vi "UHR-Fleezers Control (host) - 10.6.vi"() -> ()   [LabVIEW 2010] (continued)
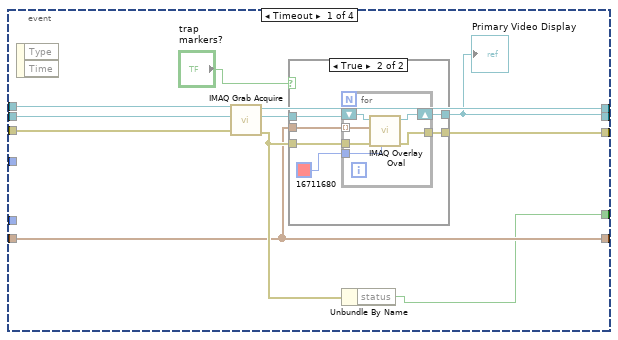
[diagram p2: hidden frame]
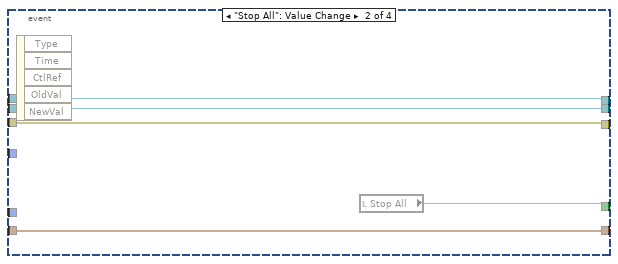
[diagram p4: hidden frame]
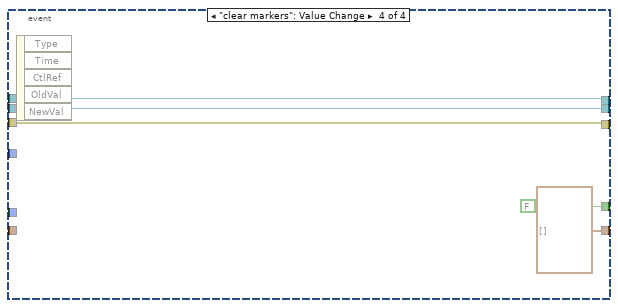
[diagram p6: hidden frame]
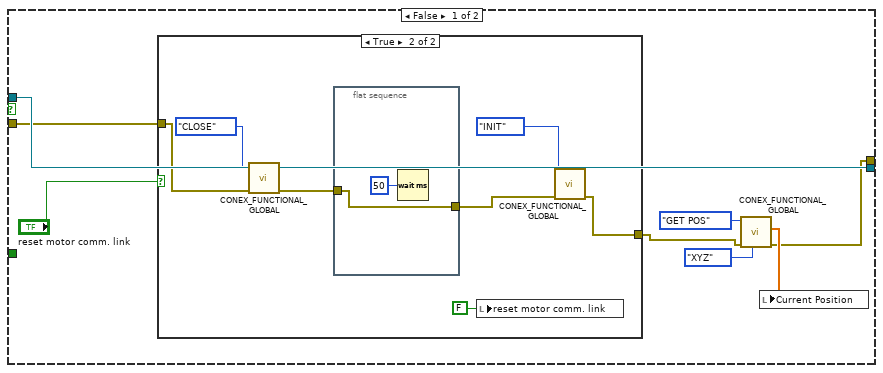
[diagram p8: hidden frame]
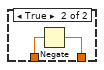
[diagram p12: hidden frame]
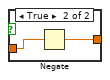
[diagram p13: hidden frame]
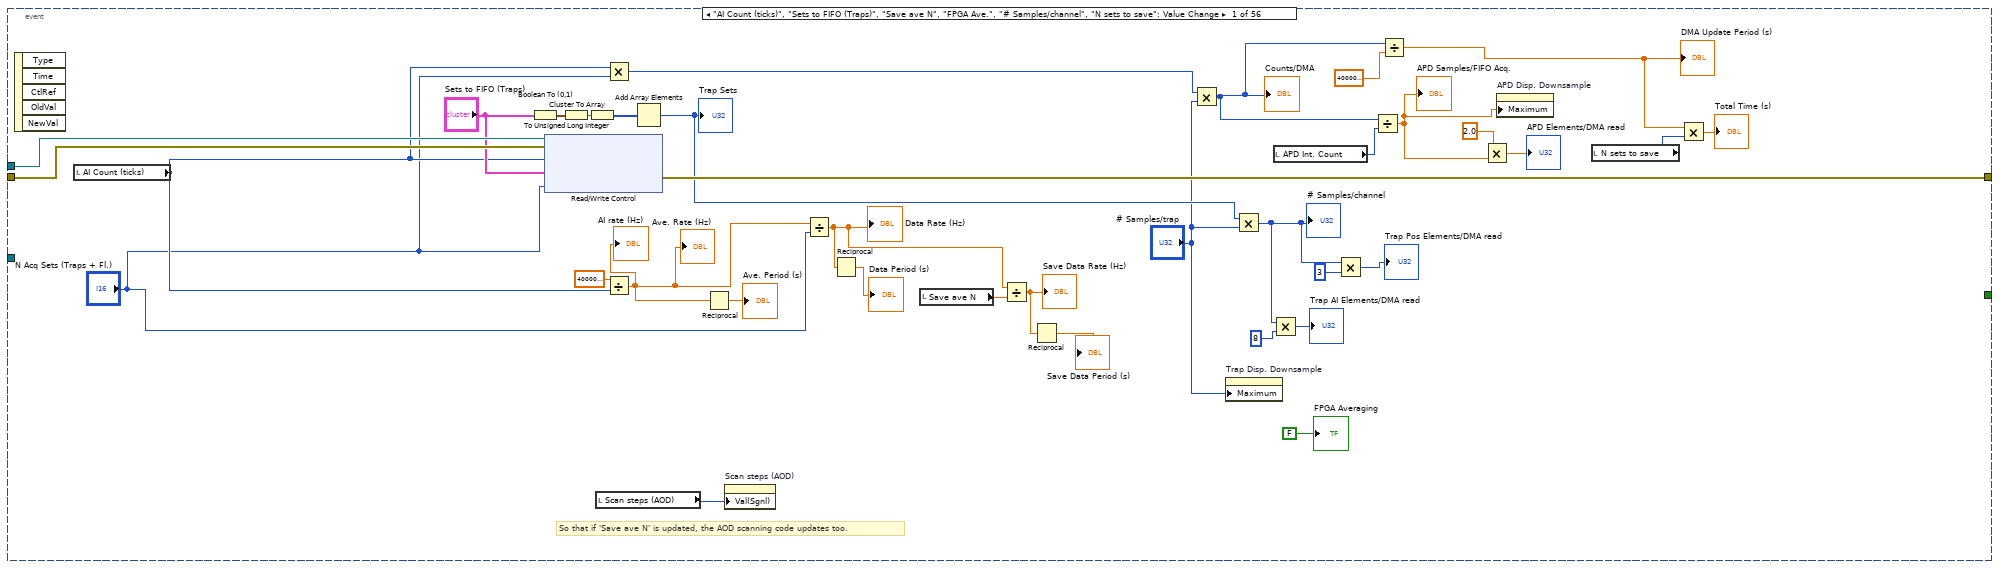
[diagram p14: hidden frame]
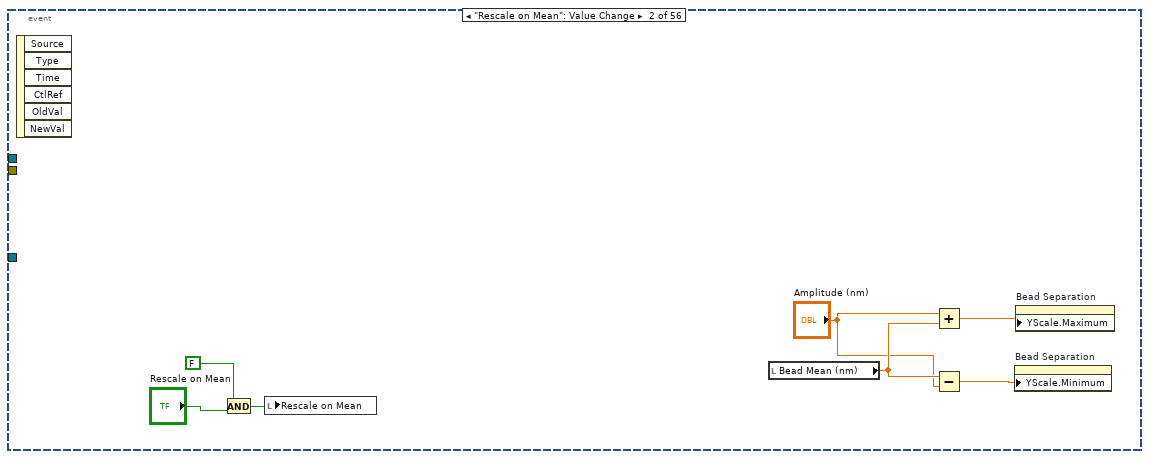
[diagram p15: hidden frame]
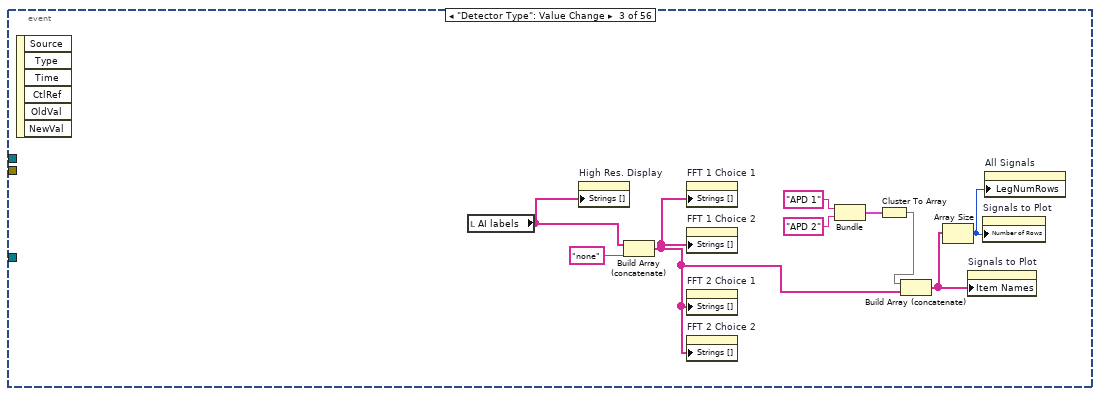
[diagram p16: hidden frame]
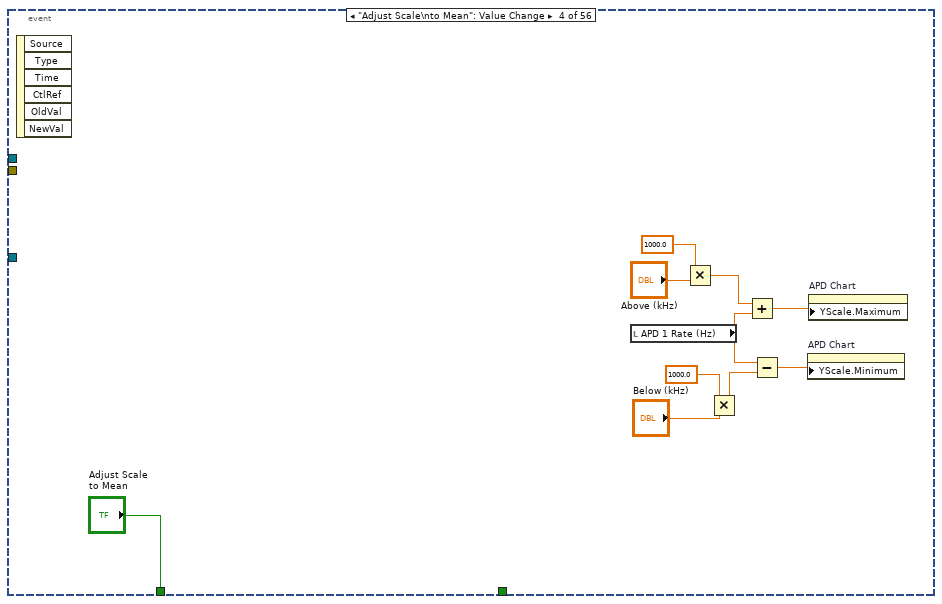
[diagram p17: hidden frame]
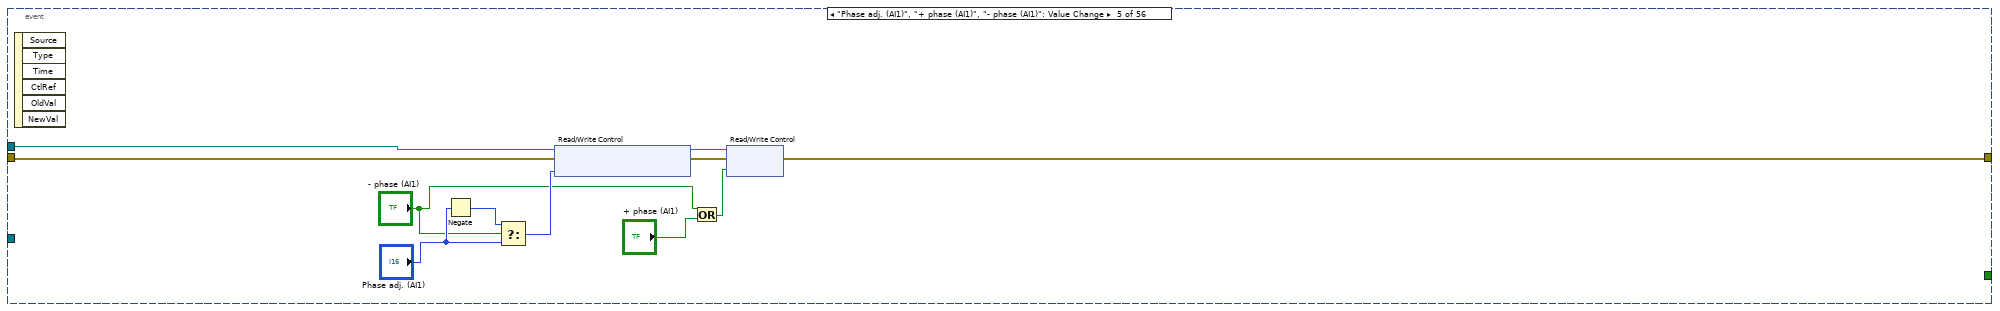
[diagram p18: hidden frame]
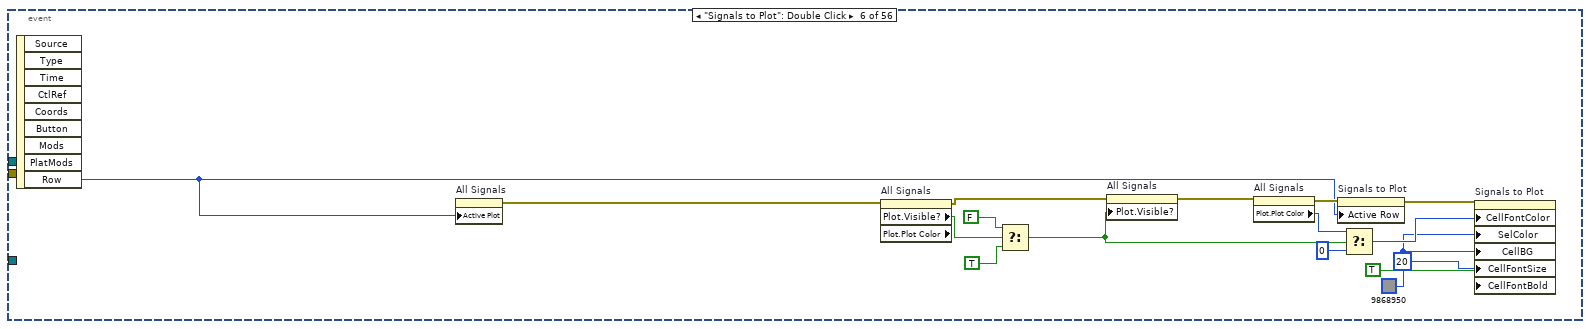
[diagram p19: hidden frame]
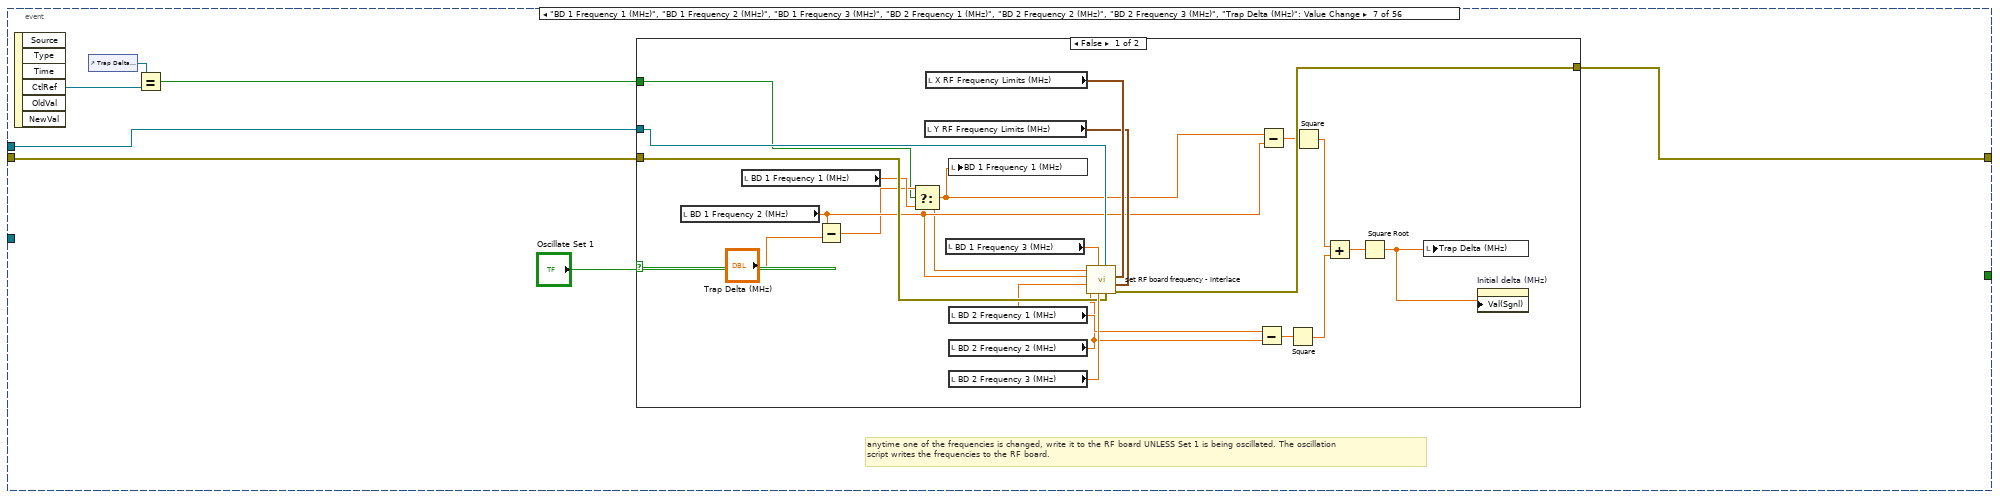
[diagram p20: hidden frame]
                n2095 = Divide "X pix/step"(x=w8753, y=w8756) -> (x/y=w8762:dbl)
                n2096 = Negate(x=w8765) -> (-x=w8766:dbl)
                n2097 = local read "Initial Y"() -> (w8772:dbl)
                n2098 = Multiply(x=w8754, y=w8763) -> (x*y=w8773:dbl)
                n2099 = Divide "X half step offset"(x=w8749, y=2.0) -> (x/y=w8759:dbl)
                n2100 = Divide "X V/pix"(x=w8749, y=w8762) -> (x/y=w8761:dbl)
                n2101 = Multiply(x=w8749, y=w8756) -> (x*y=w8768:dbl)
                n2102 = Compound Arithmetic op=ADD(w8766, w8773, w8772) -> (w8750:dbl)
                "Pointer Y (V)" <- w8750
                n2103 = Multiply(x=w8761, y=w8755) -> (x*y=w8770:dbl)
                n2104 = Negate(x=w8759) -> (-x=w8758:dbl)
                n2105 = local read "Initial X"() -> (w8771:dbl)
                n2106 = Negate(x=w8770) -> (-x=w8769:dbl)
                n2107 = Compound Arithmetic op=ADD(w8758, w8768, w8771, w8769) -> (w8751:dbl)
                "Pointer X (V)" <- w8751
                n2108 = Or(x="Set X Only", y="Set Confocal Spot (X-Y)") -> (x .or. y?=w8744:bool)
                n2109 = Or(x="Set Confocal Spot (X-Y)", y="Set Y Only") -> (x .or. y?=w8743:bool)
                n2110 = case shown="True" w8744 {
                  tunnel: w8751 -> [_ w8774]
                  frame False {
                  }
                  frame True {
                    n2111 = property on="AO2" class="Slide (strict)"("Val(Sgnl)"=w8774) -> ()  [unwired: 2 in, 2 out]
                  }
                }
                n2112 = case shown="True" w8743 {
                  tunnel: w8750 -> [_ w8775]
                  frame False {
                  }
                  frame True {
                    n2113 = property on="AO1" class="Slide (strict)"("Val(Sgnl)"=w8775) -> ()  [unwired: 2 in, 2 out]
                  }
                }
                n2114 = local write "Set Confocal Spot (X-Y)"(w8748) -> ()
                n2115 = local write "Set X Only"(w8748) -> ()
                n2116 = local write "Set Y Only"(w8748) -> ()
              }
            }
          }
          frame 3 {
            n2117 = local read "BD 2 Frequency 1 (MHz)"() -> (w8776:dbl)
            n2118 = local read "BD 1 Frequency 1 (MHz)"() -> (w8777:dbl)
            n2119 = local write "Manipulating Trap"(TRUE ("Manipulating Trap")) -> ()
            n2120 = local write "Coords"(T7 {"Horizontal"=0, "Vertical"=0} ("Coords")) -> ()
            n2121 = while {
              tunnel: w8782 -> [w8787]
              tunnel: w8780 -> [w8786]
              tunnel: w8778 -> [w8785]
              tunnel: w8777 -> [w8784]
              tunnel: w8776 -> [w8783]
              stop <- w8788 stop-if-true
              n2122 = event shown="[0] \"Pane\": Mouse Move" {
                selector: _ -> [_ _]
                dyn-events: _ -> [_ _]
                timeout: _ -> [_ _]
                tunnel: ["Force Manip Abort" w8852] -> w8788
                tunnel: w8787 -> [w8795 _]
                tunnel: w8786 -> [w8793 _]
                tunnel: w8785 -> [w8792 _]
                tunnel: w8784 -> [w8791 _]
                tunnel: w8783 -> [w8790 _]
                event Mouse Move {
                  n2123 = event-data() -> ("Time"=w8796:u32, "Coords"=w8797:T7)  [unwired: 3 out]
                  n2124 = Less?(x=w8796, y=w8795) -> (x < y?=w8794:bool)
                  n2125 = case "Makes sure old motion events prior to mouse click aren't used" shown="False" w8794 {
                    tunnel: w8797 -> [w8839 _]
                    tunnel: w8793 -> [w8840 _]
                    tunnel: w8792 -> [w8817 _]
                    tunnel: w8791 -> [w8813 _]
                    tunnel: w8790 -> [w8812 _]
                    frame False {
                      n2126 = Subtract(x=w8839, y=w8840) -> (x-y=w8838:T7)
                      "Coords" <- w8838
                      n2127 = local read "Y RF Frequency Limits (MHz)"() -> (w8798:T16)
                      n2128 = To Double Precision Float(number=w8838) -> (double precision float=w8837:cluster{"Horizontal":dbl, "Vertical":dbl})
                      n2129 = Multiply(x=cluster{"Horizontal":dbl, "Vertical":dbl} {"Horizontal"=-1.0, "Vertical"=1.0}, y="Manipulation Scaling") -> (x*y=w8833:cluster{"Horizontal":dbl, "Vertical":dbl})
                      n2130 = local read "X RF Frequency Limits (MHz)"() -> (w8799:T16)
                      n2131 = Multiply(x=w8837, y=w8833) -> (x*y=w8835:cluster{"Horizontal":dbl, "Vertical":dbl})
                      n2132 = Unbundle By Name(w8835) -> ("Horizontal"=w8830:dbl, "Vertical"=w8834:dbl)
                      n2133 = Unbundle By Name(w8798) -> ("Maximum"=w8801:dbl, "Minimum"=w8800:dbl)
                      n2134 = Boolean To (0,1)(Boolean="Manip. X?") -> (0, 1=w8828:i16)
                      n2135 = Boolean To (0,1)(Boolean="Manip. Y?") -> (0, 1=w8825:i16)
                      n2136 = local read "BD 1 Frequency 2 (MHz)"() -> (w8815:dbl)
                      n2137 = Multiply(x=w8834, y=w8825) -> (x*y=w8827:dbl)
                      n2138 = Multiply(x=w8828, y=w8830) -> (x*y=w8831:dbl)
                      n2139 = local read "BD 2 Frequency 2 (MHz)"() -> (w8814:dbl)
                      n2140 = Unbundle By Name(w8799) -> ("Maximum"=w8803:dbl, "Minimum"=w8802:dbl)
                      n2141 = Add(x=w8812, y=w8827) -> (x+y=w8805:dbl)
                      n2142 = Add(x=w8813, y=w8831) -> (x+y=w8807:dbl)
                      n2143 = In Range and Coerce(upper limit=w8803, x=w8807, lower limit=w8802) -> (coerced(x)=w8806:dbl)  [unwired: 1 out]
                      n2144 = In Range and Coerce(upper limit=w8801, x=w8805, lower limit=w8800) -> (coerced(x)=w8804:dbl)  [unwired: 1 out]
                      n2145 = Subtract(x=w8806, y=w8815) -> (x-y=w8824:dbl)
                      n2146 = Subtract(x=w8804, y=w8814) -> (x-y=w8823:dbl)
                      n2147 = Square(x=w8824) -> (x^2=w8822:dbl)
                      n2148 = Square(x=w8823) -> (x^2=w8821:dbl)
                      n2149 = Add(x=w8822, y=w8821) -> (x+y=w8820:dbl)
                      n2150 = Square Root(x=w8820) -> (sqrt(x)=w8816:dbl)
                      n2151 = In Range and Coerce(upper limit="Limit Max (MHz)", x=w8816, lower limit="Limit Min (MHz)") -> (In Range?=w8809:bool)  [unwired: 1 out]
                      n2152 = Not(x="Limits Enable") -> (.not. x?=w8808:bool)
                      n2153 = Or(x=w8809, y=w8808) -> (x .or. y?=w8810:bool)
                      n2154 = case shown="True" w8810 {
                        tunnel: w8817 -> [_ w8850]
                        tunnel: w8816 -> [_ w8841]
                        tunnel: w8806 -> [_ w8848]
                        tunnel: w8815 -> [_ w8847]
                        tunnel: w8804 -> [_ w8846]
                        tunnel: w8814 -> [_ w8845]
                        tunnel: w8799 -> [_ w8843]
                        tunnel: w8798 -> [_ w8842]
                        frame False {
                        }
                        frame True {
                          n2155 = local read "BD 1 Frequency 3 (MHz)"() -> (w8849:dbl)
                          n2156 = local read "BD 2 Frequency 3 (MHz)"() -> (w8844:dbl)
                          n2157 = local write "Trap Delta (MHz)"(w8841) -> ()
                          n2158 = property on="Initial delta (MHz)" class="DigNum (strict)"("Val(Sgnl)"=w8841) -> ()  [unwired: 2 in, 2 out]
                          n2159 = call "set RF board frequency - interlace.vi"("Board 2 Frequency Limits"=w8842, "Board 1 Frequency Limits"=w8843, "FPGA VI Reference In"=w8850, "Board 2 Frequency 3 (MHz)"=w8844, "Board 1 Frequency 3 (MHz)"=w8849, "Board 2 Frequency 2 (MHz)"=w8845, "Board 2 Frequency 1 (MHz)"=w8846, "Board 1 Frequency 2 (MHz)"=w8847, "Board 1 Frequency 1  (MHz)"=w8848) -> ()  [unwired: 1 in, 2 out]
                          n2160 = local write "BD 2 Frequency 1 (MHz)"(w8846) -> ()
                          n2161 = local write "BD 1 Frequency 1 (MHz)"(w8848) -> ()
                        }
                      }
                    }
                    frame True {
                    }
                  }
                }
                event Mouse Up {
                  n2162 = event-data() -> ("Button"=w8851:u16)  [unwired: 8 out]
                  n2163 = case shown="3" w8851 {
                    tunnel: [FALSE TRUE] -> w8852
                    frame 0, Default {
                    }
                    frame 3 {
                      n2164 = local write "Manipulating Trap"(FALSE ("Manipulating Trap")) -> ()
                    }
                  }
                }
              }
            }
          }
        }
      }
      event Mouse Move {
        n2165 = event-data() -> ()  [unwired: 6 out]
      }
    }
    n2166 = local read "Stop All"() -> (w8673:bool)
    n2167 = node-c288() -> ()  [unwired: 2 out]
  }
  n2168 = timed-loop "Oscillate AOD (debugging)" {
    tunnel: w18 -> [w8857]
    tunnel: [w8856] -> w35
    timing: w79 -> [_]
    timing-out: [_] -> w78
    stop <- w8856 stop-if-true
    n2169 = node-c288() -> ()  [unwired: 2 out]
    n2170 = event shown="[0] \"Oscillate Set 1\", \"Fish for Tether\": Value Change" {
      selector: _ -> [_ _ _]
      dyn-events: _ -> [_ _ _]
      timeout: _ -> [_ _ _]
      tunnel: w8857 -> [w8864 _ _]
      tunnel: [FALSE ("Stop All") _ w9133] -> w8856
      event "Oscillate Set 1", "Fish for Tether": Value Change {
        n2171 = event-data() -> ()  [unwired: 6 out]
        n2172 = local read "Oscillate Set 1"() -> (w8863:bool)
        n2173 = Or(x=w8863, y="Fish for Tether") -> (x .or. y?=w8861:bool)
        n2174 = case shown="True" w8861 {
          tunnel: w8864 -> [_ w8867]
          tunnel: "Fish for Tether" -> [_ w8866]
          frame False {
          }
          frame True {
            n2175 = case shown="False" w8866 {
              frame False {
              }
              frame True {
                n2176 = local write "Scan axis 2"(TRUE) -> ()
                n2177 = local write "Tether"(FALSE ("Tether")) -> ()
              }
            }
            n2178 = node-c288("Period") -> (w8869:T26)  [unwired: 3 out]
            n2179 = timed-loop "Oscillate AOD" {
              timing: w8869 -> [_]
              timing-out: [_] -> w8868
              tunnel: w8867 -> [w8879]
              tunnel: w8866 -> [w8878]
              i -> [w8881]
              stop <- w8877 stop-if-true
              n2180 = node-c288() -> (w8880:i64)  [unwired: 1 out]
              n2181 = flat-sequence {
                tunnel: w8881 -> [w8908]
                tunnel: w8880 -> [w8907]
                tunnel: w8879 -> [w8888]
                tunnel: w8878 -> [w8891]
                tunnel: [w8891] -> w8876
                tunnel: [w8890] -> w8875
                tunnel: [w8887] -> w8874
                tunnel: [w8884] -> w8872
                tunnel: w8876 -> [w8944]
                tunnel: w8875 -> [w8942]
                tunnel: w8874 -> [w8941]
                tunnel: [w8940] -> w8873
                tunnel: w8872 -> [w8939]
                tunnel: [w9008] -> w8877
                tunnel: w8873 -> [w9006]
                frame #0 {
                  n2182 = Divide(x=w8907, y=i64 1000) -> (x/y=w8902:dbl)
                  n2183 = Multiply(x=w8902, y=w8908) -> (x*y=w8904:dbl)
                  n2184 = Multiply(x="Osc. freq. (Hz)", y=6.283185307179586) -> (x*y=w8905:dbl)
                  n2185 = Multiply(x=w8905, y=w8904) -> (x*y=w8886:dbl)
                  n2186 = local read "BD 1 Frequency 2 (MHz)"() -> (w8889:dbl)
                  n2187 = local read "BD 1 Frequency 1 (MHz)"() -> (w8882:dbl)
                  n2188 = case shown="True" w8891 {
                    tunnel: w8886 -> [w8914 w8920]
                    tunnel: w8889 -> [_ w8931]
                    tunnel: [w8911 w8926] -> w8892
                    tunnel: [FALSE w8923] -> w8887
                    tunnel: [0.0 w8916] -> w8884
                    tunnel: w8882 -> [_ w8915]
                    frame False {
                      n2189 = Sine(x=w8914) -> (sin(x)=w8912:dbl)
                      n2190 = Multiply(x=w8912, y="Osc. amp. (MHz)") -> (x*y=w8911:dbl)
                    }
                    frame True {
                      n2191 = Cosine(x=w8920) -> (cos(x)=w8934:dbl)
                      n2192 = Subtract(x=w8931, y=w8915) -> (x-y=w8930:dbl)
                      n2193 = Decrement(x=w8934) -> (x-1=w8933:dbl)
                      n2194 = Subtract(x=w8930, y="Closest Delta (MHz)") -> (x-y=w8927:dbl)
                      n2195 = Divide(x=w8933, y=-2.0) -> (x/y=w8928:dbl)
                      n2196 = Multiply(x=w8928, y=w8927) -> (x*y=w8926:dbl)
                      n2197 = local read "Vec Mean of T1 T2"() -> (w8922:dbl[])
                      n2198 = Greater?(x=w8922, y="Stop F (pN)") -> (0:w8924:bool[])
                      n2199 = Or Array Elements(Boolean array=w8924) -> (logical OR=w8923:bool)
                      n2200 = Divide(x=w8920, y=6.283185307179586) -> (x/y=w8919:dbl)
                      n2201 = Round Toward +Infinity(x=w8919) -> (ceil(x): smallest int >= x=w8916:dbl)
                      "Attempts" <- w8916
                      n2202 = Greater?(x=w8916, y="Attempt Limit") -> (0:w8918:bool)
                      n2203 = case shown="True" w8918 {
                        frame False {
                        }
                        frame True {
                          n2204 = local write "Fish for Tether"(FALSE ("Fish for Tether")) -> ()
                          n2205 = call <vilib>:"Beep.vi"() -> ()  [unwired: 3 in, 9 out]
                          n2206 = local read "Messages"() -> (w8936:string)
                          n2207 = call "Update messages.vi"("Message to add"="Tether fishing timeout." ("Messages"), "Old message string"=w8936) -> ("New message string"=→"Messages":string)
                        }
                      }
                    }
                  }
                  n2208 = local read "BD 2 Frequency 1 (MHz)"() -> (w8893:dbl)
                  n2209 = Select(t=w8882, s="Scan axis 2", f=w8893) -> (s? t:f=w8896:dbl)
                  n2210 = Add(x=w8892, y=w8896) -> (x+y=w8890:dbl)
                  n2211 = Select(t=w8890, s="Scan axis 2", f=w8882) -> (s? t:f=w8883:dbl)
                  n2212 = Select(t=w8893, s="Scan axis 2", f=w8890) -> (s? t:f=w8898:dbl)
                  n2213 = local read "Y RF Frequency Limits (MHz)"() -> (w8894:T16)
                  n2214 = local read "X RF Frequency Limits (MHz)"() -> (w8895:T16)
                  n2215 = local read "BD 1 Frequency 3 (MHz)"() -> (w8901:dbl)
                  n2216 = local read "BD 2 Frequency 2 (MHz)"() -> (w8900:dbl)
                  n2217 = local read "BD 2 Frequency 3 (MHz)"() -> (w8899:dbl)
                  n2218 = call "set RF board frequency - interlace.vi"("Board 2 Frequency Limits"=w8894, "Board 1 Frequency Limits"=w8895, "FPGA VI Reference In"=w8888, "Board 2 Frequency 3 (MHz)"=w8899, "Board 1 Frequency 3 (MHz)"=w8901, "Board 2 Frequency 2 (MHz)"=w8900, "Board 2 Frequency 1 (MHz)"=w8898, "Board 1 Frequency 2 (MHz)"=w8889, "Board 1 Frequency 1  (MHz)"=w8883) -> ()  [unwired: 1 in, 2 out]
                }
                frame #1 {
                  n2219 = And(x=w8944, y=w8941) -> (x .and. y?=w8943:bool)
                  n2220 = case "Only if were fishing and now formed tether" shown="False" w8943 {
                    tunnel: w8942 -> [w8946 w8958]
                    tunnel: [w8945 w8957] -> w8940
                    tunnel: w8939 -> [_ w8953]
                    frame False {
                      n2221 = local read "Fish for Tether"() -> (w8945:bool)
                      n2222 = case shown="True" w8945 {
                        tunnel: w8946 -> [_ _]
                        frame False {
                        }
                        frame True {
                        }
                      }
                    }
                    frame True {
                      w8957 = FALSE ("Fish for Tether")
                      n2223 = call <vilib>:"Beep.vi"() -> ()  [unwired: 3 in, 9 out]
                      n2224 = Number To Decimal String(number=w8953, width (-)=i16 1) -> (decimal integer string=w8951:string)
                      n2225 = case shown="\"1\", Default" "Then..." {
                        selector: "Then..." -> [_ w8961]
                        tunnel: w8958 -> [w8960 _]
                        frame "1", Default {
                          n2226 = property on="BD 1 Frequency 1 (MHz)" class="DigNum (strict)"("Val(Sgnl)"=w8960) -> ()  [unwired: 2 in, 2 out]
                        }
                        frame "2", "3", "4", "5", "6" {
                          n2227 = flat-sequence {
                            tunnel: w8961 -> [w8963]
                            frame #0 {
                              n2228 = property on="Trap Delta (MHz)" class="DigNum (strict)"("Val(Sgnl)"="Move to Delta 1 (MHz)") -> ()  [unwired: 2 in, 2 out]
                            }
                            frame #1 {
                              n2229 = case shown="\"5\", \"6\"" w8963 {
                                selector: w8963 -> [w8966 w8976 _]
                                frame "3", "4" {
                                n2230 = flat-sequence {
                                tunnel: w8966 -> [w8967]
                                tunnel: [w8967] -> w8964
                                tunnel: [w8969] -> w8965
                                tunnel: w8964 -> [w8969]
                                tunnel: w8965 -> [w8973]
                                frame #0 {
                                n2231 = property on="Green Laser ON/Interlacing" class="Bool (strict)"("Val(Sgnl)"=TRUE ("Value (Signaling)")) -> ()  [unwired: 2 in, 2 out]
                                }
                                frame #1 {
                                n2232 = Multiply(x="Wait Before Save (s)", y=u32 1000 ("x")) -> (x*y=w8971:u32)
                                n2233 = Wait (ms)(milliseconds to wait=w8971) -> ()  [unwired: 1 out]
                                }
                                frame #2 {
                                n2234 = property on="Start Saving" class="Bool (strict)"("Value"=TRUE ("Start Saving")) -> ()  [unwired: 2 in, 2 out]
                                n2235 = case shown="\"4\"" w8973 {
                                frame Default {
                                }
                                frame "4" {
                                n2236 = property on="Fl. Triggered..." class="Bool (strict)"("Val(Sgnl)"=TRUE ("Value (Signaling)")) -> ()  [unwired: 2 in, 2 out]
                                }
                                }
                                }
                                }
                                }
                                frame "5", "6" {
                                n2237 = stacked-sequence {
                                tunnel: w8976 -> [_ _ _ _ _ _ _ _ w8993 _ _]
                                frame #0 {
                                n2238 = Replace Array Subset(array=u32[] [0] ("Index Values"), new element="Raster Set Upon Tether", index=0) -> (w8977:u32[])
                                n2239 = property on="Saved AOD Raster Scan Parameter Sets" class="Arr (strict)"("Index Values"=w8977) -> ()  [unwired: 2 in, 2 out]
                                }
                                frame #1 {
                                n2240 = Wait (ms)(milliseconds to wait=u32 500) -> ()  [unwired: 1 out]
                                }
                                frame #2 {
                                n2241 = property on="Load parameters" class="Bool (strict)"("Val(Sgnl)"=TRUE ("Value (Signaling)")) -> ()  [unwired: 2 in, 2 out]
                                }
                                frame #3 {
                                n2242 = Wait (ms)(milliseconds to wait=u32 500) -> ()  [unwired: 1 out]
                                }
                                frame #4 {
                                n2243 = property on="Trap Raster Scan" class="Bool (strict)"("Val(Sgnl)"=TRUE ("Value (Signaling)")) -> ()  [unwired: 2 in, 2 out]
                                }
                                frame #5 {
                                n2244 = Wait (ms)(milliseconds to wait=u32 2000) -> ()  [unwired: 1 out]
                                }
                                frame #6 {
                                n2245 = while {
                                stop <- w8988 stop-if-true
                                n2246 = local read "Raster Scanning..."() -> (w8987:bool)
                                n2247 = local read "Saving..."() -> (w8990:bool)
                                n2248 = Wait (ms)(milliseconds to wait=u32 100) -> ()  [unwired: 1 out]
                                n2249 = Not(x=w8990) -> (.not. x?=w8989:bool)
                                n2250 = Not(x=w8987) -> (.not. x?=w8986:bool)
                                n2251 = And(x=w8989, y=w8986) -> (x .and. y?=w8988:bool)
                                }
                                }
                                frame #7 {
                                n2252 = property on="Trap Delta (MHz)" class="DigNum (strict)"("Val(Sgnl)"="Move to Delta 2 (MHz)") -> ()  [unwired: 2 in, 2 out]
                                }
                                frame #8 {
                                n2253 = local read "Tether"() -> (w8994:bool)
                                n2254 = case shown="True" w8994 {
                                tunnel: w8993 -> [_ w8995]
                                frame False {
                                }
                                frame True {
                                n2255 = flat-sequence {
                                tunnel: w8995 -> [w8997]
                                frame #0 {
                                n2256 = Wait (ms)(milliseconds to wait=u32 500) -> ()  [unwired: 1 out]
                                }
                                frame #1 {
                                n2257 = case shown="\"6\"" w8997 {
                                frame Default {
                                }
                                frame "6" {
                                n2258 = property on="Green Laser ON/Interlacing" class="Bool (strict)"("Val(Sgnl)"=TRUE ("Green Laser ON/Interlacing")) -> ()  [unwired: 2 in, 2 out]
                                }
                                }
                                }
                                frame #2 {
                                n2259 = Wait (ms)(milliseconds to wait=u32 500) -> ()  [unwired: 1 out]
                                }
                                frame #3 {
                                n2260 = local write "Start Saving"("Save at end (5, 6)") -> ()
                                }
                                }
                                }
                                }
                                }
                                frame #9 {
                                n2261 = local read "Bead Sep. Int. Time (s)"() -> (w9003:dbl)
                                n2262 = Multiply(x=w9003, y=1000.0) -> (x*y=w9002:dbl)
                                n2263 = Wait (ms)(milliseconds to wait=w9002) -> ()  [unwired: 1 out]
                                }
                                frame #10 {
                                n2264 = property on="Rescale on Mean" class="Bool (strict)"("Val(Sgnl)"=TRUE ("Value (Signaling)")) -> ()  [unwired: 2 in, 2 out]
                                }
                                }
                                }
                                frame "2", Default {
                                }
                              }
                            }
                          }
                        }
                      }
                      n2265 = Concatenate Strings("Formed tether in ", w8951, " attempt(s)." ("string")) -> (w8948:string)
                      n2266 = local read "Messages"() -> (w8955:string)
                      n2267 = local write "Fish for Tether"(w8957) -> ()
                      n2268 = call "Update messages.vi"("Message to add"=w8948, "Old message string"=w8955) -> ("New message string"=w8954:string)
                      n2269 = local write "Messages"(w8954) -> ()
                      n2270 = Get Date/Time In Seconds() -> (seconds since 1Jan1904=→"Time tether formed":timestamp)
                      "Tether" <- "Tether Alarm?"
                    }
                  }
                }
                frame #2 {
                  n2271 = local read "Oscillate Set 1"() -> (w9007:bool)
                  n2272 = local read "Stop All"() -> (w9009:bool)
                  n2273 = Not Or(1:w9006, 2:w9007) -> (0:w9005:bool)
                  n2274 = Compound Arithmetic op=OR(w9009, w9005) -> (w9008:bool)
                }
              }
              n2275 = node-c288() -> ()  [unwired: 2 out]
            }
            n2276 = node-c288(w8868) -> ()  [unwired: 1 out]
          }
        }
      }
      event "Fl. Triggered...": Value Change {
        n2277 = event-data() -> ()  [unwired: 7 out]
        n2278 = case shown="True" "Fl. Triggered..." {
          frame False {
          }
          frame True {
            n2279 = node-c288() -> (w9021:T26)  [unwired: 4 out]
            n2280 = timed-loop {
              timing: w9021 -> [_]
              timing-out: [_] -> w9020
              tunnel: "Action" -> [w9025]
              shift-right: [w9022] -> _
              shift-left: u8 255 -> [w9024]
              stop <- w9026 stop-if-true
              n2281 = node-c288() -> ()  [unwired: 2 out]
              n2282 = flat-sequence {
                tunnel: w9025 -> [w9038]
                tunnel: w9024 -> [w9035]
                tunnel: [w9034] -> w9023
                tunnel: [w9124] -> w9026
                tunnel: w9023 -> [w9123]
                tunnel: [w9123] -> w9022
                frame #0 {
                  n2283 = local read "Delta Fl. 2"() -> (w9029:dbl)
                  n2284 = local read "Delta Fl. 1"() -> (w9030:dbl)
                  n2285 = Select(t=w9030, s="APD to Watch", f=w9029) -> (s? t:f=w9028:dbl)
                  n2286 = Multiply(x="Fl. Delta Thresh. (kHz)", y=1000.0) -> (x*y=w9037:dbl)
                  n2287 = Greater?(x=w9028, y=w9037) -> (0:w9032:bool)
                  n2288 = Or(x="Force Yank", y=w9032) -> (x .or. y?=w9033:bool)
                  n2289 = case shown="True" w9033 {
                    tunnel: w9038 -> [_ w9048]
                    tunnel: w9035 -> [w9040 w9044]
                    tunnel: [w9040 w9041] -> w9034
                    frame False {
                    }
                    frame True {
                      n2290 = flat-sequence {
                        tunnel: w9045 -> [w9054]
                        tunnel: [w9054] -> w9049
                        tunnel: w9048 -> [w9053]
                        tunnel: [w9053] -> w9047
                        tunnel: [w9052] -> w9046
                        tunnel: w9044 -> [w9051]
                        tunnel: [w9050] -> w9043
                        tunnel: w9049 -> [w9079]
                        tunnel: w9047 -> [w9078]
                        tunnel: w9046 -> [w9077]
                        tunnel: w9043 -> [w9076]
                        tunnel: [w9076] -> w9042
                        tunnel: w9042 -> [w9121]
                        tunnel: [w9121] -> w9041
                        frame #0 {
                          n2291 = call <vilib>:"Beep.vi"() -> ()  [unwired: 3 in, 9 out]
                          n2292 = local write "Waiting"(FALSE ("Waiting")) -> ()
                          n2293 = Increment(x=w9051) -> (x+1=w9050:u8)
                          n2294 = case shown="\"Yank\"" w9053 {
                            tunnel: w9050 -> [_ _ w9060]
                            frame "Image" {
                              n2295 = property on="Confocal Image" class="Bool (strict)"("Val(Sgnl)"=TRUE ("Value (Signaling)")) -> ()  [unwired: 2 in, 2 out]
                            }
                            frame "Alarm", Default {
                            }
                            frame "Yank" {
                              n2296 = flat-sequence {
                                tunnel: w9060 -> [w9063]
                                tunnel: [w9062] -> w9059
                                tunnel: ["N Array El"] -> w9058
                                tunnel: w9059 -> [w9073]
                                tunnel: w9058 -> [w9069]
                                frame #0 {
                                n2297 = Multiply(x="Yank Delay (s)", y=1000.0) -> (x*y=w9066:dbl)
                                n2298 = Quotient & Remainder(x=w9063, y="N Array El") -> (x-y*floor(x/y)=w9062:u8)  [unwired: 1 out]
                                n2299 = Wait (ms)(milliseconds to wait=w9066) -> ()  [unwired: 1 out]
                                }
                                frame #1 {
                                n2300 = Random Number (0-1)() -> (number: 0 to 1=w9070:dbl)
                                n2301 = Multiply(x=w9069, y=w9070) -> (x*y=w9068:dbl)
                                n2302 = Round Toward -Infinity(1:w9068) -> (0:w9067:dbl)
                                n2303 = Select(t=w9067, s="Random Choice", f=w9073) -> (s? t:f=w9071:dbl)
                                n2304 = Index Array(array="Yank to Delta Array (MHz)", index=w9071) -> (element=w9074:dbl)
                                n2305 = property on="Trap Delta (MHz)" class="DigNum (strict)"("Val(Sgnl)"=w9074) -> ()  [unwired: 2 in, 2 out]
                                }
                              }
                            }
                          }
                          n2306 = local read "Time (s)"() -> (w9052:dbl)
                          "Fl. High" <- TRUE ("Yanking")
                        }
                        frame #1 {
                          n2307 = node-c288() -> (w9081:T26)  [unwired: 4 out]
                          n2308 = timed-loop {
                            timing: w9081 -> [_]
                            timing-out: [_] -> w9080
                            tunnel: w9079 -> [w9097]
                            tunnel: w9078 -> [w9095]
                            tunnel: w9077 -> [w9094]
                            stop <- w9096 stop-if-true
                            n2309 = node-c288() -> ()  [unwired: 2 out]
                            n2310 = local read "Fl. Delta Thresh. (kHz)"() -> (w9089:dbl)
                            n2311 = local read "Fl. Triggered..."() -> (w9098:bool)
                            n2312 = local read "Delta Fl. 1"() -> (w9085:dbl)
                            n2313 = local read "Delta Fl. 2"() -> (w9083:dbl)
                            n2314 = local read "Stop All"() -> (w9092:bool)
                            n2315 = local read "APD to Watch"() -> (w9084:bool)
                            n2316 = Select(t=w9085, s=w9084, f=w9083) -> (s? t:f=w9082:dbl)
                            n2317 = Not(x=w9098) -> (.not. x?=w9093:bool)
                            n2318 = Multiply(x=w9089, y=1000.0) -> (x*y=w9088:dbl)
                            n2319 = Negate(x=w9088) -> (-x=w9087:dbl)
                            n2320 = Less?(x=w9082, y=w9087) -> (x < y?=w9091:bool)
                            n2321 = Compound Arithmetic op=OR(w9091, w9092, w9093, "Force Reset") -> (w9096:bool)
                            n2322 = case shown="True" w9096 {
                              tunnel: w9097 -> [_ w9109]
                              tunnel: w9095 -> [_ w9108]
                              tunnel: w9094 -> [_ w9106]
                              frame False {
                              }
                              frame True {
                                n2323 = case shown="\"Yank\"" w9108 {
                                tunnel: w9109 -> [_ w9110]
                                frame "Image", Default {
                                }
                                frame "Yank" {
                                n2324 = flat-sequence {
                                tunnel: [w9115] -> w9111
                                tunnel: w9110 -> [w9115]
                                tunnel: w9111 -> [w9116]
                                frame #0 {
                                n2325 = local read "Yank Delay (s)"() -> (w9114:dbl)
                                n2326 = Multiply(x=w9114, y=1000.0) -> (x*y=w9112:dbl)
                                n2327 = Wait (ms)(milliseconds to wait=w9112) -> ()  [unwired: 1 out]
                                }
                                frame #1 {
                                n2328 = property on="Trap Delta (MHz)" class="DigNum (strict)"("Val(Sgnl)"=w9116) -> ()  [unwired: 2 in, 2 out]
                                }
                                }
                                }
                                }
                                n2329 = local read "Time (s)"() -> (w9107:dbl)
                                n2330 = Subtract(x=w9107, y=w9106) -> (x-y=w9103:dbl)
                                "Duration (s)" <- w9103
                                n2331 = Number To Decimal String(number=w9103, width (-)=i16 0) -> (decimal integer string=w9101:string)
                                n2332 = Concatenate Strings(w9101, " s fluorescence event." ("string")) -> (w9099:string)
                                n2333 = local read "Messages"() -> (w9105:string)
                                n2334 = call "Update messages.vi"("Message to add"=w9099, "Old message string"=w9105) -> ("New message string"=w9104:string)
                                n2335 = call <vilib>:"Beep.vi"() -> ()  [unwired: 3 in, 9 out]
                                n2336 = local write "Messages"(w9104) -> ()
                              }
                            }
                            n2337 = node-c288() -> ()  [unwired: 2 out]
                          }
                          n2338 = node-c288(w9080) -> ()  [unwired: 1 out]
                        }
                        frame #2 {
                          n2339 = local write "Fl. High"(FALSE ("Yanking")) -> ()
                        }
                      }
                      n2340 = local read "Trap Delta (MHz)"() -> (w9045:dbl)
                    }
                  }
                }
                frame #1 {
                  n2341 = local read "Stop All"() -> (w9127:bool)
                  n2342 = local read "Fl. Triggered..."() -> (w9125:bool)
                  n2343 = Not(x=w9125) -> (.not. x?=w9126:bool)
                  n2344 = Or(x=w9126, y=w9127) -> (x .or. y?=w9124:bool)
                  n2345 = Not(x=w9124) -> (.not. x?=→"Waiting":bool)
                }
              }
              n2346 = node-c288() -> ()  [unwired: 2 out]
            }
            n2347 = node-c288(w9020) -> ()  [unwired: 1 out]
          }
        }
      }
      event "Stop All": Value Change {
        n2348 = event-data() -> ()  [unwired: 7 out]
        n2349 = local read "Stop All"() -> (w9133:bool)
      }
    }
    n2350 = node-c288() -> ()  [unwired: 2 out]
  }
  n2351 = node-c288(w5) -> ()  [unwired: 1 out]
  n2352 = call-poly <vilib>:"Close Input Device.vi"("device ID"=w23) -> ()  [unwired: 9 in, 1 out]
  n2353 = node-c288(w8) -> ()  [unwired: 1 out]
  n2354 = call "hamilton_controller.vi"("error in"=w2, "action"=T17."DISCONNECT") -> ()  [unwired: 9 in, 1 out]
  n2355 = node-c288(w80) -> ()  [unwired: 1 out]
  n2356 = node-c288(w73) -> ()  [unwired: 1 out]
  n2357 = node-c288(w78) -> ()  [unwired: 1 out]
  n2358 = node-c288(w168) -> ()  [unwired: 1 out]
  n2359 = flat-sequence {
    tunnel: w32 -> [w9138]
    tunnel: [w9137] -> w38
    tunnel: [w9134] -> w37
    tunnel: w36 -> [_]
    tunnel: w35 -> [_]
    tunnel: w34 -> [_]
    tunnel: w33 -> [_]
    tunnel: w31 -> [w9135]
    tunnel: w38 -> [w9200]
    tunnel: w37 -> [w9199]
    frame #0 {
      w9136 = FALSE ("APD to FIFO")
      n2360 = xnode "Read/Write Control"("FPGA VI Reference In"=w9138, "error in"=w9135, "APD to FIFO"=w9136, "AI to FIFO"=w9136) -> ("FPGA VI Reference Out"=w9137:T20, "error out"=w9134:errorcluster)
    }
    frame #1 {
      n2361 = xnode "Invoke Method"("FPGA VI Reference In"=w9200, "error in"=w9199) -> ("FPGA VI Reference Out"=w9198:T20)  [unwired: 1 out]
      n2362 = xnode "Close FPGA VI Reference"("FPGA VI Reference In"=w9198) -> ()  [unwired: 1 in, 1 out]
    }
  }
